vi "FlexMag - 23-03-2023.vi"() -> ()   [LabVIEW 2018] (continued)
                          n16847 = Less Or Equal?(x=w21889, y=0.2) -> (x <= y?=w21887:bool)
                          n16848 = case shown="True" w21887 {
                            tunnel: [FALSE TRUE] -> w21891
                            frame False {
                              n16849 = Wait Until Next ms Multiple(millisecond multiple=u32 200) -> ()  [unwired: 1 out]
                            }
                            frame True {
                            }
                          }
                          n16850 = local read "ch3 pumpdown alg"() -> (w21896:bool)
                          n16851 = local read "abort ch3"() -> (w21894:bool)
                          n16852 = Not(x=w21896) -> (.not. x?=w21895:bool)
                          n16853 = Compound Arithmetic op=OR(w21891, w21894, w21895) -> (w21897:bool)
                        }
                      }
                      frame True {
                      }
                    }
                  }
                }
              }
              frame #31 {
                # "tp start"
                n16854 = local read "ch3 pumpdown alg"() -> (w21903:bool)
                n16855 = case shown="True" w21903 {
                  frame False {
                  }
                  frame True {
                    n16856 = local read "abort ch3"() -> (w21904:bool)
                    n16857 = case shown="False" w21904 {
                      frame False {
                        n16858 = stacked-sequence {
                          frame #0 {
                            n16859 = flat-sequence {
                              frame #0 {
                                n16860 = local write "Tp3 auto start"(TRUE ("Tp1 auto start")) -> ()
                                n16861 = Wait (ms)(milliseconds to wait=u32 100) -> ()  [unwired: 1 out]
                              }
                              frame #1 {
                                n16862 = Wait (ms)(milliseconds to wait=u32 2000) -> ()  [unwired: 1 out]
                              }
                              frame #2 {
                                n16863 = disable-structure shown="Disabled" {
                                frame Disabled {
                                n16864 = local write "Tp1 Start initial"(TRUE ("Tp1 Start initial")) -> ()
                                }
                                frame Enabled {
                                }
                                }
                              }
                              frame #3 {
                                n16865 = Wait (ms)(milliseconds to wait=u32 2000) -> ()  [unwired: 1 out]
                              }
                              frame #4 {
                                n16866 = local write "Tp3 auto low speed"(TRUE ("Tp1 auto start")) -> ()
                                n16867 = Wait (ms)(milliseconds to wait=u32 100) -> ()  [unwired: 1 out]
                              }
                            }
                          }
                          frame #1 {
                            n16868 = while {
                              i -> [w21920]
                              stop <- w21914 stop-if-true
                              # "200 sec ?"
                              n16869 = Greater Or Equal?(x=w21920, y=1000) -> (x >= y?=w21913:bool)
                              n16870 = case shown="True" w21913 {
                                frame False {
                                }
                                frame True {
                                n16871 = local write "Warning Message"("CH3 PumpDown process  is canceled !\nCH3 TP couldn't be started" ("Warning Message")) -> ()
                                n16872 = local write "ch3 pumpdown error"(TRUE ("ch1 pumpdown error")) -> ()
                                }
                              }
                              n16873 = local read "ch3 pumpdown alg"() -> (w21917:bool)
                              n16874 = local read "ch3_tp_gui"() -> (w21912:bool)
                              n16875 = local read "abort ch3"() -> (w21915:bool)
                              n16876 = Not(x=w21917) -> (.not. x?=w21916:bool)
                              n16877 = Wait Until Next ms Multiple(millisecond multiple=u32 200) -> ()  [unwired: 1 out]
                              n16878 = Compound Arithmetic op=OR(w21912, w21915, w21916) -> (w21914:bool)
                            }
                          }
                        }
                      }
                      frame True {
                      }
                    }
                  }
                }
              }
              frame #32 {
                n16879 = local read "ch3 pumpdown alg"() -> (w21923:bool)
                n16880 = case shown="True" w21923 {
                  frame False {
                  }
                  frame True {
                    n16881 = local read "abort ch3"() -> (w21924:bool)
                    n16882 = case shown="False" w21924 {
                      frame False {
                        n16883 = local write "ch3 tp start led"(TRUE ("ch1 tp start led")) -> ()
                        n16884 = Wait (ms)(milliseconds to wait=u32 1000) -> ()  [unwired: 1 out]
                      }
                      frame True {
                      }
                    }
                  }
                }
              }
              frame #33 {
                n16885 = local read "ch3 pumpdown alg"() -> (w21927:bool)
                n16886 = case shown="True" w21927 {
                  frame False {
                  }
                  frame True {
                    n16887 = local read "abort ch3"() -> (w21928:bool)
                    n16888 = case shown="False" w21928 {
                      frame False {
                        n16889 = while {
                          i -> [w21935]
                          stop <- w21939 stop-if-true
                          # "30 min"
                          n16890 = Greater?(x=w21935, y=9000) -> (0:w21932:bool)
                          n16891 = case shown="True" w21932 {
                            frame False {
                            }
                            frame True {
                              n16892 = local write "Warning Message"("CH3 PumpDown process  is canceled !\nCH3 CH Pressure couldn't reach under 0.01 Torr" ("Warning Message")) -> ()
                              n16893 = local write "ch3 pumpdown error"(TRUE ("ch1 pumpdown error")) -> ()
                            }
                          }
                          n16894 = local read "ch3 ch pg torr"() -> (w21931:dbl)
                          n16895 = Less Or Equal?(x=w21931, y=0.09) -> (x <= y?=w21929:bool)
                          n16896 = case shown="False" w21929 {
                            tunnel: [FALSE TRUE] -> w21933
                            frame False {
                              n16897 = Wait Until Next ms Multiple(millisecond multiple=u32 200) -> ()  [unwired: 1 out]
                            }
                            frame True {
                            }
                          }
                          n16898 = local read "ch3 pumpdown alg"() -> (w21938:bool)
                          n16899 = local read "abort ch3"() -> (w21936:bool)
                          n16900 = Not(x=w21938) -> (.not. x?=w21937:bool)
                          n16901 = Compound Arithmetic op=OR(w21933, w21936, w21937) -> (w21939:bool)
                        }
                      }
                      frame True {
                      }
                    }
                  }
                }
              }
              frame #34 {
                n16902 = local read "ch3 pumpdown alg"() -> (w21945:bool)
                n16903 = case shown="True" w21945 {
                  frame False {
                  }
                  frame True {
                    n16904 = local read "abort ch3"() -> (w21946:bool)
                    n16905 = case shown="False" w21946 {
                      frame False {
                        n16906 = local write "ch3 ch press under 0.01 T led"(TRUE ("ch1 pressure under 0.05 torr led")) -> ()
                        n16907 = Wait (ms)(milliseconds to wait=u32 1000) -> ()  [unwired: 1 out]
                      }
                      frame True {
                      }
                    }
                  }
                }
              }
              frame #35 {
                n16908 = local read "ch3 pumpdown alg"() -> (w21949:bool)
                n16909 = case shown="True" w21949 {
                  frame False {
                  }
                  frame True {
                    n16910 = local read "abort ch3"() -> (w21950:bool)
                    n16911 = case shown="False" w21950 {
                      frame False {
                        n16912 = stacked-sequence {
                          frame #0 {
                            n16913 = while {
                              i -> [w21955]
                              stop <- w21959 stop-if-true
                              n16914 = Greater?(x=w21955, y=200) -> (0:w21952:bool)
                              n16915 = case shown="True" w21952 {
                                frame False {
                                }
                                frame True {
                                n16916 = local write "Warning Message"("CH3 PumpDown process  is canceled !\nCH3 CC couldn't be opened" ("Warning Message")) -> ()
                                n16917 = local write "ch3 pumpdown error"(TRUE ("ch1 pumpdown error")) -> ()
                                }
                              }
                              n16918 = local read "CH3_CC_DI"() -> (w21951:bool)
                              n16919 = case shown="False" w21951 {
                                tunnel: [FALSE TRUE] -> w21953
                                frame False {
                                n16920 = Wait Until Next ms Multiple(millisecond multiple=u32 200) -> ()  [unwired: 1 out]
                                n16921 = local write "CH3_CC_DO"(TRUE ("CH1_CC_DO")) -> ()
                                }
                                frame True {
                                }
                              }
                              n16922 = local read "ch3 pumpdown alg"() -> (w21958:bool)
                              n16923 = local read "abort ch3"() -> (w21956:bool)
                              n16924 = Not(x=w21958) -> (.not. x?=w21957:bool)
                              n16925 = Compound Arithmetic op=OR(w21953, w21956, w21957) -> (w21959:bool)
                            }
                          }
                          frame #1 {
                            n16926 = while {
                              i -> [w21968]
                              stop <- w21970 stop-if-true
                              n16927 = local read "ch3 pumpdown alg"() -> (w21971:bool)
                              n16928 = local read "abort ch3"() -> (w21973:bool)
                              n16929 = Greater Or Equal?(x=w21968, y=300) -> (x >= y?=w21966:bool)
                              n16930 = Not(x=w21971) -> (.not. x?=w21972:bool)
                              n16931 = Compound Arithmetic op=OR(w21966, w21973, w21972) -> (w21970:bool)
                              n16932 = Wait Until Next ms Multiple(millisecond multiple=u32 200) -> ()  [unwired: 1 out]
                            }
                          }
                        }
                      }
                      frame True {
                      }
                    }
                  }
                }
              }
              frame #36 {
                n16933 = local read "ch3 pumpdown alg"() -> (w21974:bool)
                n16934 = case shown="True" w21974 {
                  frame False {
                  }
                  frame True {
                    n16935 = local read "abort ch3"() -> (w21975:bool)
                    n16936 = case shown="False" w21975 {
                      frame False {
                        n16937 = local write "ch3 cc open led"(TRUE ("ch1 ch cc open led")) -> ()
                        n16938 = Wait (ms)(milliseconds to wait=u32 1000) -> ()  [unwired: 1 out]
                      }
                      frame True {
                      }
                    }
                  }
                }
              }
              frame #37 {
                n16939 = local read "ch3 pumpdown alg"() -> (w21978:bool)
                n16940 = case shown="True" w21978 {
                  frame False {
                  }
                  frame True {
                    n16941 = local read "abort ch3"() -> (w21979:bool)
                    n16942 = case shown="False" w21979 {
                      frame False {
                        n16943 = while {
                          i -> [w21990]
                          stop <- w21994 stop-if-true
                          # "60 min"
                          n16944 = Multiply(x=27000 ("y"), y=3) -> (x*y=w21980:i32)
                          n16945 = Greater?(x=w21990, y=w21980) -> (0:w21988:bool)
                          n16946 = case shown="True" w21988 {
                            frame False {
                            }
                            frame True {
                              n16947 = local write "Warning Message"("CH3 PumpDown process  is canceled !\nCH3 CH Pressure couldn't reach to desired pressure" ("Warning Message")) -> ()
                              n16948 = local write "ch3 pumpdown error"(TRUE ("ch1 pumpdown error")) -> ()
                            }
                          }
                          n16949 = local read "ch3 cc torr"() -> (w21987:dbl)
                          n16950 = Multiply(x=0.75, y="ch3 desired pressure") -> (x*y=w21983:dbl)
                          n16951 = Less Or Equal?(x=w21987, y=w21983) -> (x <= y?=w21986:bool)
                          n16952 = case shown="True" w21986 {
                            tunnel: [FALSE TRUE] -> w21989
                            frame False {
                              n16953 = Wait Until Next ms Multiple(millisecond multiple=u32 200) -> ()  [unwired: 1 out]
                            }
                            frame True {
                            }
                          }
                          n16954 = local read "ch3 pumpdown alg"() -> (w21993:bool)
                          n16955 = local read "abort ch3"() -> (w21991:bool)
                          n16956 = Not(x=w21993) -> (.not. x?=w21992:bool)
                          n16957 = Compound Arithmetic op=OR(w21989, w21991, w21992) -> (w21994:bool)
                        }
                      }
                      frame True {
                      }
                    }
                  }
                }
              }
              frame #38 {
                n16958 = local read "ch3 pumpdown alg"() -> (w22000:bool)
                n16959 = case shown="True" w22000 {
                  frame False {
                  }
                  frame True {
                    n16960 = local read "abort ch3"() -> (w22001:bool)
                    n16961 = case shown="False" w22001 {
                      frame False {
                        n16962 = local write "ch3 desired pressure led"(TRUE ("ch1 pumdown completed led")) -> ()
                        n16963 = Wait (ms)(milliseconds to wait=u32 1000) -> ()  [unwired: 1 out]
                      }
                      frame True {
                      }
                    }
                  }
                }
              }
              frame #39 {
                n16964 = local read "ch3 pumpdown alg"() -> (w22004:bool)
                n16965 = case shown="True" w22004 {
                  frame False {
                  }
                  frame True {
                    n16966 = local read "abort ch3"() -> (w22005:bool)
                    n16967 = case shown="False" w22005 {
                      frame False {
                        w22007 = TRUE ("Buzzer DO")
                        n16968 = local write "Buzzer DO"(w22007) -> ()
                        n16969 = local write "ch3 pd completed led"(w22007) -> ()
                        n16970 = Wait (ms)(milliseconds to wait=u32 3000) -> ()  [unwired: 1 out]
                        n16971 = local write "CH3_BG_BV_DO"(TRUE ("CH1_BG_BV_DO")) -> ()
                        n16972 = local write "System Status"("CH3 PUMPDOWN PROCESS COMPLETED" ("System Status")) -> ()
                      }
                      frame True {
                      }
                    }
                  }
                }
              }
              frame #40 {
                n16973 = local read "ch3 pumpdown alg"() -> (w22010:bool)
                n16974 = case shown="True" w22010 {
                  frame False {
                  }
                  frame True {
                    n16975 = local read "abort ch3"() -> (w22011:bool)
                    n16976 = case shown="False" w22011 {
                      frame False {
                        w22013 = FALSE ("Buzzer DO")
                        n16977 = local write "Buzzer DO"(w22013) -> ()
                        n16978 = local write "ch3 pumpdown alg"(w22013) -> ()
                        n16979 = local write "Pump Down CH3"(w22013) -> ()
                        n16980 = Wait (ms)(milliseconds to wait=u32 3000) -> ()  [unwired: 1 out]
                        n16981 = local write "System Status"("SEMI-AUTOMATIC MODE " ("System Status")) -> ()
                      }
                      frame True {
                      }
                    }
                  }
                }
              }
            }
          }
          frame True {
          }
        }
      }
    }
    n16982 = case shown="True" "ch3 shutdown alg" {
      frame False {
      }
      frame True {
        n16983 = local read "abort ch3"() -> (w21094:bool)
        n16984 = case shown="False" w21094 {
          frame False {
            n16985 = stacked-sequence {
              frame #0 {
                n16986 = stacked-sequence {
                  frame #0 {
                    n16987 = local write "ch3 vent?"(FALSE ("ch1 vent?")) -> ()
                    n16988 = Wait (ms)(milliseconds to wait=u32 1000) -> ()  [unwired: 1 out]
                  }
                  frame #1 {
                    n16989 = local write "System Status"("CH3 SHUTDOWN PROCESS IN PROGRESS" ("System Status")) -> ()
                  }
                  frame #2 {
                    n16990 = Two Button Dialog(message="Do you want to Vent CH3 ?", 1:"No, SHUTDOWN only" ("F button name (\"Cancel\")"), 2:"Yes, VENT! CH3" ("T button name (\"OK\")")) -> (T button?=w21098:bool)
                    "ch3 vent?" <- w21098
                    n16991 = case shown="True" w21098 {
                      frame False {
                      }
                      frame True {
                        w21102 = FALSE ("CH2_Trns_BP_Right_DO")
                        n16992 = local write "CH2_Trns_BP_Left_DO"(w21102) -> ()
                        n16993 = local write "CH4_Trns_BP_Right_DO"(w21102) -> ()
                      }
                    }
                  }
                }
              }
              frame #1 {
                # "ATMs close"
                n16994 = local read "ch3 shutdown alg"() -> (w21103:bool)
                n16995 = case shown="True" w21103 {
                  frame False {
                  }
                  frame True {
                    n16996 = local read "abort ch3"() -> (w21104:bool)
                    n16997 = case shown="False" w21104 {
                      frame False {
                        w21105 = FALSE ("CH1_PL_ATM_DO")
                        n16998 = local write "CH3_PL_ATM_DO"(w21105) -> ()
                        n16999 = local write "CH3_CH_ATM_DO"(w21105) -> ()
                        n17000 = Wait (ms)(milliseconds to wait=u32 3000) -> ()  [unwired: 1 out]
                      }
                      frame True {
                      }
                    }
                  }
                }
              }
              frame #2 {
                n17001 = local read "ch3 shutdown alg"() -> (w21107:bool)
                n17002 = case shown="True" w21107 {
                  frame False {
                  }
                  frame True {
                    n17003 = local read "abort ch3"() -> (w21108:bool)
                    n17004 = case shown="False" w21108 {
                      frame False {
                        n17005 = local write "ch3 sd atms close led"(TRUE ("ch1 sd cc close led")) -> ()
                        n17006 = Wait (ms)(milliseconds to wait=u32 1000) -> ()  [unwired: 1 out]
                      }
                      frame True {
                      }
                    }
                  }
                }
              }
              frame #3 {
                # "CC close"
                n17007 = local read "ch3 shutdown alg"() -> (w21111:bool)
                n17008 = case shown="True" w21111 {
                  frame False {
                  }
                  frame True {
                    n17009 = local read "abort ch3"() -> (w21112:bool)
                    n17010 = case shown="False" w21112 {
                      frame False {
                        n17011 = while {
                          i -> [w21117]
                          stop <- w21121 stop-if-true
                          n17012 = Greater?(x=w21117, y=100) -> (0:w21114:bool)
                          n17013 = case shown="True" w21114 {
                            frame False {
                            }
                            frame True {
                              n17014 = local write "Warning Message"("CH3 ShutDown process  is canceled !\nCH3 CC couldn't be closed" ("Warning Message")) -> ()
                              n17015 = local write "ch3 shutdown error"(TRUE ("ch1 pumpdown error")) -> ()
                            }
                          }
                          n17016 = local read "CH3_CC_DI"() -> (w21113:bool)
                          n17017 = case shown="True" w21113 {
                            tunnel: [TRUE FALSE] -> w21115
                            frame False {
                            }
                            frame True {
                              n17018 = Wait Until Next ms Multiple(millisecond multiple=u32 200) -> ()  [unwired: 1 out]
                              n17019 = local write "CH3_CC_DO"(FALSE ("CH1_CC_DO")) -> ()
                            }
                          }
                          n17020 = local read "ch3 shutdown alg"() -> (w21120:bool)
                          n17021 = local read "abort ch3"() -> (w21118:bool)
                          n17022 = Not(x=w21120) -> (.not. x?=w21119:bool)
                          n17023 = Compound Arithmetic op=OR(w21115, w21118, w21119) -> (w21121:bool)
                        }
                      }
                      frame True {
                      }
                    }
                  }
                }
              }
              frame #4 {
                n17024 = local read "ch3 shutdown alg"() -> (w21128:bool)
                n17025 = case shown="True" w21128 {
                  frame False {
                  }
                  frame True {
                    n17026 = local read "abort ch3"() -> (w21129:bool)
                    n17027 = case shown="False" w21129 {
                      frame False {
                        n17028 = local write "ch3 sd cc close led"(TRUE ("ch1 sd cc close led")) -> ()
                        n17029 = Wait (ms)(milliseconds to wait=u32 1000) -> ()  [unwired: 1 out]
                      }
                      frame True {
                      }
                    }
                  }
                }
              }
              frame #5 {
                # "bg bv close"
                n17030 = local read "ch3 shutdown alg"() -> (w21132:bool)
                n17031 = case shown="True" w21132 {
                  frame False {
                  }
                  frame True {
                    n17032 = local read "abort ch3"() -> (w21133:bool)
                    n17033 = case shown="False" w21133 {
                      frame False {
                        n17034 = while {
                          i -> [w21138]
                          stop <- w21142 stop-if-true
                          n17035 = Greater?(x=w21138, y=100) -> (0:w21135:bool)
                          n17036 = case shown="True" w21135 {
                            frame False {
                            }
                            frame True {
                              n17037 = local write "Warning Message"("CH3 ShutDown process  is canceled !\nCH3 BG BV couldn't be closed" ("Warning Message")) -> ()
                              n17038 = local write "ch3 shutdown error"(TRUE ("ch1 pumpdown error")) -> ()
                            }
                          }
                          n17039 = local read "CH3_BG_BV_DI"() -> (w21134:bool)
                          n17040 = case shown="True" w21134 {
                            tunnel: [TRUE FALSE] -> w21136
                            frame False {
                            }
                            frame True {
                              n17041 = Wait Until Next ms Multiple(millisecond multiple=u32 200) -> ()  [unwired: 1 out]
                              n17042 = local write "CH3_BG_BV_DO"(FALSE ("CH1_CC_DO")) -> ()
                            }
                          }
                          n17043 = local read "ch3 shutdown alg"() -> (w21141:bool)
                          n17044 = local read "abort ch3"() -> (w21139:bool)
                          n17045 = Not(x=w21141) -> (.not. x?=w21140:bool)
                          n17046 = Compound Arithmetic op=OR(w21136, w21139, w21140) -> (w21142:bool)
                        }
                      }
                      frame True {
                      }
                    }
                  }
                }
              }
              frame #6 {
                n17047 = local read "ch3 shutdown alg"() -> (w21149:bool)
                n17048 = case shown="True" w21149 {
                  frame False {
                  }
                  frame True {
                    n17049 = local read "abort ch3"() -> (w21150:bool)
                    n17050 = case shown="False" w21150 {
                      frame False {
                        n17051 = local write "ch3 sd bg bv close led"(TRUE ("ch1 sd cc close led")) -> ()
                        n17052 = Wait (ms)(milliseconds to wait=u32 1000) -> ()  [unwired: 1 out]
                      }
                      frame True {
                      }
                    }
                  }
                }
              }
              frame #7 {
                # "TP stop"
                n17053 = local read "ch3 shutdown alg"() -> (w21153:bool)
                n17054 = case shown="True" w21153 {
                  frame False {
                  }
                  frame True {
                    n17055 = local read "abort ch3"() -> (w21154:bool)
                    n17056 = case shown="False" w21154 {
                      frame False {
                        n17057 = stacked-sequence {
                          frame #0 {
                            n17058 = flat-sequence {
                              frame #0 {
                                n17059 = local write "Tp3 auto stop"(TRUE ("Tp1 auto stop")) -> ()
                                n17060 = Wait (ms)(milliseconds to wait=u32 100) -> ()  [unwired: 1 out]
                              }
                              frame #1 {
                                n17061 = Wait (ms)(milliseconds to wait=u32 5000) -> ()  [unwired: 1 out]
                              }
                              frame #2 {
                                n17062 = local write "Tp3 auto stop"(TRUE ("Tp1 auto stop")) -> ()
                                n17063 = Wait (ms)(milliseconds to wait=u32 100) -> ()  [unwired: 1 out]
                              }
                            }
                          }
                          frame #1 {
                            n17064 = while {
                              i -> [w21171]
                              stop <- w21166 stop-if-true
                              n17065 = Multiply(x=3000 ("y"), y=5) -> (x*y=w21161:i32)
                              n17066 = Greater Or Equal?(x=w21171, y=w21161) -> (x >= y?=w21165:bool)
                              n17067 = case shown="True" w21165 {
                                frame False {
                                }
                                frame True {
                                n17068 = local write "Warning Message"("CH3 ShutDown process  is canceled !\nCH3 TP couldn't be stopped" ("Warning Message")) -> ()
                                n17069 = local write "ch3 shutdown error"(TRUE ("ch1 pumpdown error")) -> ()
                                }
                              }
                              n17070 = local read "ch3 shutdown alg"() -> (w21169:bool)
                              n17071 = local read "ch3_tp_gui"() -> (w21164:bool)
                              n17072 = local read "abort ch3"() -> (w21167:bool)
                              n17073 = Not(x=w21164) -> (.not. x?=w21163:bool)
                              n17074 = Not(x=w21169) -> (.not. x?=w21168:bool)
                              n17075 = Wait Until Next ms Multiple(millisecond multiple=u32 200) -> ()  [unwired: 1 out]
                              n17076 = Compound Arithmetic op=OR(w21163, w21167, w21168) -> (w21166:bool)
                            }
                          }
                        }
                      }
                      frame True {
                      }
                    }
                  }
                }
              }
              frame #8 {
                n17077 = local read "ch3 shutdown alg"() -> (w21174:bool)
                n17078 = case shown="True" w21174 {
                  frame False {
                  }
                  frame True {
                    n17079 = local read "abort ch3"() -> (w21175:bool)
                    n17080 = case shown="False" w21175 {
                      frame False {
                        n17081 = local write "ch3 sd tp stop led"(TRUE ("ch1 sd cc close led")) -> ()
                        n17082 = Wait (ms)(milliseconds to wait=u32 1000) -> ()  [unwired: 1 out]
                      }
                      frame True {
                      }
                    }
                  }
                }
              }
              frame #9 {
                # "tp bv close"
                n17083 = local read "ch3 shutdown alg"() -> (w21178:bool)
                n17084 = case shown="True" w21178 {
                  frame False {
                  }
                  frame True {
                    n17085 = local read "abort ch3"() -> (w21179:bool)
                    n17086 = case shown="False" w21179 {
                      frame False {
                        n17087 = while {
                          i -> [w21184]
                          stop <- w21188 stop-if-true
                          n17088 = Greater?(x=w21184, y=100) -> (0:w21181:bool)
                          n17089 = case shown="True" w21181 {
                            frame False {
                            }
                            frame True {
                              n17090 = local write "Warning Message"("CH3 ShutDown process  is canceled !\nCH3 TP BV couldn't be closed" ("Warning Message")) -> ()
                              n17091 = local write "ch3 shutdown error"(TRUE ("ch1 pumpdown error")) -> ()
                            }
                          }
                          n17092 = local read "CH3_TP_BV_DI"() -> (w21180:bool)
                          n17093 = case shown="True" w21180 {
                            tunnel: [TRUE FALSE] -> w21182
                            frame False {
                            }
                            frame True {
                              n17094 = Wait Until Next ms Multiple(millisecond multiple=u32 200) -> ()  [unwired: 1 out]
                              n17095 = local write "CH3_TP_BV_DO"(FALSE ("CH1_CC_DO")) -> ()
                            }
                          }
                          n17096 = local read "ch3 shutdown alg"() -> (w21187:bool)
                          n17097 = local read "abort ch3"() -> (w21185:bool)
                          n17098 = Not(x=w21187) -> (.not. x?=w21186:bool)
                          n17099 = Compound Arithmetic op=OR(w21182, w21185, w21186) -> (w21188:bool)
                        }
                      }
                      frame True {
                      }
                    }
                  }
                }
              }
              frame #10 {
                n17100 = local read "ch3 shutdown alg"() -> (w21195:bool)
                n17101 = case shown="True" w21195 {
                  frame False {
                  }
                  frame True {
                    n17102 = local read "abort ch3"() -> (w21196:bool)
                    n17103 = case shown="False" w21196 {
                      frame False {
                        n17104 = local write "ch3 sd tp bv close led"(TRUE ("ch1 sd cc close led")) -> ()
                        n17105 = Wait (ms)(milliseconds to wait=u32 1000) -> ()  [unwired: 1 out]
                      }
                      frame True {
                      }
                    }
                  }
                }
              }
              frame #11 {
                # "mp stop"
                n17106 = local read "ch3 shutdown alg"() -> (w21199:bool)
                n17107 = case shown="True" w21199 {
                  frame False {
                  }
                  frame True {
                    n17108 = local read "abort ch3"() -> (w21200:bool)
                    n17109 = case shown="False" w21200 {
                      frame False {
                        n17110 = while {
                          i -> [w21205]
                          stop <- w21209 stop-if-true
                          n17111 = Greater?(x=w21205, y=100) -> (0:w21202:bool)
                          n17112 = case shown="True" w21202 {
                            frame False {
                            }
                            frame True {
                              n17113 = local write "Warning Message"("CH3 ShutDown process  is canceled !\nCH3 MP couldn't be stopped" ("Warning Message")) -> ()
                              n17114 = local write "ch3 shutdown error"(TRUE ("ch1 pumpdown error")) -> ()
                            }
                          }
                          n17115 = local read "CH3_MP_DI"() -> (w21201:bool)
                          n17116 = case shown="True" w21201 {
                            tunnel: [TRUE FALSE] -> w21203
                            frame False {
                            }
                            frame True {
                              n17117 = Wait Until Next ms Multiple(millisecond multiple=u32 200) -> ()  [unwired: 1 out]
                              n17118 = local write "CH3_MP_DO"(FALSE ("CH1_CC_DO")) -> ()
                            }
                          }
                          n17119 = local read "ch3 shutdown alg"() -> (w21208:bool)
                          n17120 = local read "abort ch3"() -> (w21206:bool)
                          n17121 = Not(x=w21208) -> (.not. x?=w21207:bool)
                          n17122 = Compound Arithmetic op=OR(w21203, w21206, w21207) -> (w21209:bool)
                        }
                      }
                      frame True {
                      }
                    }
                  }
                }
              }
              frame #12 {
                n17123 = local read "ch3 shutdown alg"() -> (w21216:bool)
                n17124 = case shown="True" w21216 {
                  frame False {
                  }
                  frame True {
                    n17125 = local read "abort ch3"() -> (w21217:bool)
                    n17126 = case shown="False" w21217 {
                      frame False {
                        n17127 = local write "ch3 sd mp stop led"(TRUE ("ch1 sd cc close led")) -> ()
                        n17128 = Wait (ms)(milliseconds to wait=u32 1000) -> ()  [unwired: 1 out]
                      }
                      frame True {
                      }
                    }
                  }
                }
              }
              frame #13 {
                # "pl vbv open"
                n17129 = local read "ch3 shutdown alg"() -> (w21220:bool)
                n17130 = case shown="True" w21220 {
                  frame False {
                  }
                  frame True {
                    n17131 = local read "abort ch3"() -> (w21221:bool)
                    n17132 = case shown="False" w21221 {
                      frame False {
                        n17133 = while {
                          i -> [w21226]
                          stop <- w21230 stop-if-true
                          n17134 = Greater?(x=w21226, y=100) -> (0:w21223:bool)
                          n17135 = case shown="True" w21223 {
                            frame False {
                            }
                            frame True {
                              n17136 = local write "Warning Message"("CH3 ShutDown process  is canceled !\nCH3 PL VBV couldn't be opened" ("Warning Message")) -> ()
                              n17137 = local write "ch3 shutdown alg"(TRUE ("ch1 pumpdown error")) -> ()
                            }
                          }
                          n17138 = local read "CH3_PL_VBV_DI"() -> (w21222:bool)
                          n17139 = case shown="False" w21222 {
                            tunnel: [FALSE TRUE] -> w21224
                            frame False {
                              n17140 = Wait Until Next ms Multiple(millisecond multiple=u32 200) -> ()  [unwired: 1 out]
                              n17141 = local write "CH3_PL_VBV_DO"(TRUE ("CH1_CC_DO")) -> ()
                            }
                            frame True {
                            }
                          }
                          n17142 = local read "ch3 shutdown alg"() -> (w21229:bool)
                          n17143 = local read "abort ch3"() -> (w21227:bool)
                          n17144 = Not(x=w21229) -> (.not. x?=w21228:bool)
                          n17145 = Compound Arithmetic op=OR(w21224, w21227, w21228) -> (w21230:bool)
                        }
                      }
                      frame True {
                      }
                    }
                  }
                }
              }
              frame #14 {
                n17146 = local read "ch3 shutdown alg"() -> (w21237:bool)
                n17147 = case shown="True" w21237 {
                  frame False {
                  }
                  frame True {
                    n17148 = local read "abort ch3"() -> (w21238:bool)
                    n17149 = case shown="False" w21238 {
                      frame False {
                        n17150 = local write "ch3 sd pl vbv open led"(TRUE ("ch1 sd cc close led")) -> ()
                        n17151 = Wait (ms)(milliseconds to wait=u32 1000) -> ()  [unwired: 1 out]
                      }
                      frame True {
                      }
                    }
                  }
                }
              }
              frame #15 {
                n17152 = local read "ch3 shutdown alg"() -> (w21241:bool)
                n17153 = case shown="True" w21241 {
                  frame False {
                  }
                  frame True {
                    n17154 = local read "abort ch3"() -> (w21242:bool)
                    n17155 = case shown="False" w21242 {
                      frame False {
                        n17156 = local read "ch3 vent?"() -> (w21243:bool)
                        n17157 = case shown="False" w21243 {
                          frame False {
                            n17158 = stacked-sequence {
                              frame #0 {
                                n17159 = local read "ch3 shutdown alg"() -> (w21244:bool)
                                n17160 = case shown="True" w21244 {
                                frame False {
                                }
                                frame True {
                                n17161 = flat-sequence {
                                frame #0 {
                                n17162 = local write "pcgv3 auto close"(TRUE ("pcgv1 auto open")) -> ()
                                }
                                frame #1 {
                                n17163 = Wait (ms)(milliseconds to wait=u32 2000) -> ()  [unwired: 1 out]
                                }
                                frame #2 {
                                n17164 = local write "pcgv3 auto close"(TRUE ("pcgv1 auto open")) -> ()
                                }
                                }
                                }
                                }
                              }
                              frame #1 {
                                n17165 = while {
                                i -> [w21255]
                                stop <- w21251 stop-if-true
                                n17166 = Greater Or Equal?(x=w21255, y=200) -> (x >= y?=w21257:bool)
                                n17167 = case shown="True" w21257 {
                                frame False {
                                }
                                frame True {
                                n17168 = local write "ch3 shutdown error"(TRUE ("ch1 pumpdown error")) -> ()
                                n17169 = local write "Warning Message"("CH3 ShutDown process  is canceled !\nCH3 PC GV couldn't be closed" ("Warning Message")) -> ()
                                }
                                }
                                n17170 = local read "ch3_pcgv_gui"() -> (w21248:bool)
                                n17171 = local read "abort ch3"() -> (w21252:bool)
                                n17172 = local read "ch3 shutdown alg"() -> (w21254:bool)
                                n17173 = Wait Until Next ms Multiple(millisecond multiple=u32 200) -> ()  [unwired: 1 out]
                                n17174 = Not(x=w21248) -> (.not. x?=w21249:bool)
                                n17175 = Not(x=w21254) -> (.not. x?=w21253:bool)
                                n17176 = Compound Arithmetic op=OR(w21249, w21252, w21253) -> (w21251:bool)
                                }
                              }
                            }
                          }
                          frame True {
                            n17177 = stacked-sequence {
                              frame #0 {
                                n17178 = local read "ch3 shutdown alg"() -> (w21260:bool)
                                n17179 = case shown="True" w21260 {
                                frame False {
                                }
                                frame True {
                                n17180 = flat-sequence {
                                frame #0 {
                                n17181 = local write "pcgv3 auto open"(TRUE ("pcgv1 auto open")) -> ()
                                }
                                frame #1 {
                                n17182 = Wait (ms)(milliseconds to wait=u32 2000) -> ()  [unwired: 1 out]
                                }
                                frame #2 {
                                n17183 = local write "pcgv3 auto open"(TRUE ("pcgv1 auto open")) -> ()
                                }
                                }
                                }
                                }
                              }
                              frame #1 {
                                n17184 = while {
                                i -> [w21270]
                                stop <- w21266 stop-if-true
                                n17185 = Greater Or Equal?(x=w21270, y=200) -> (x >= y?=w21272:bool)
                                n17186 = case shown="True" w21272 {
                                frame False {
                                }
                                frame True {
                                n17187 = local write "ch3 shutdown error"(TRUE ("ch1 pumpdown error")) -> ()
                                n17188 = local write "Warning Message"("CH3 ShutDown process  is canceled !\nCH3 PC GV couldn't be opened" ("Warning Message")) -> ()
                                }
                                }
                                n17189 = local read "ch3 shutdown alg"() -> (w21269:bool)
                                n17190 = local read "ch3_pcgv_gui"() -> (w21265:bool)
                                n17191 = local read "abort ch3"() -> (w21267:bool)
                                n17192 = Wait Until Next ms Multiple(millisecond multiple=u32 200) -> ()  [unwired: 1 out]
                                n17193 = Not(x=w21269) -> (.not. x?=w21268:bool)
                                n17194 = Compound Arithmetic op=OR(w21265, w21267, w21268) -> (w21266:bool)
                                }
                              }
                            }
                          }
                        }
                      }
                      frame True {
                      }
                    }
                  }
                }
              }
              frame #16 {
                n17195 = local read "ch3 shutdown alg"() -> (w21275:bool)
                n17196 = case shown="True" w21275 {
                  frame False {
                  }
                  frame True {
                    n17197 = local read "abort ch3"() -> (w21276:bool)
                    n17198 = case shown="False" w21276 {
                      frame False {
                        n17199 = local read "ch3 vent?"() -> (w21277:bool)
                        n17200 = case shown="False" w21277 {
                          frame False {
                            n17201 = local write "ch3 sd pcgv close led"(TRUE ("ch1 sd cc close led")) -> ()
                            n17202 = Wait (ms)(milliseconds to wait=u32 1000) -> ()  [unwired: 1 out]
                          }
                          frame True {
                            n17203 = local write "ch3 sd pcgv open led"(TRUE ("ch1 sd cc close led")) -> ()
                            n17204 = Wait (ms)(milliseconds to wait=u32 1000) -> ()  [unwired: 1 out]
                          }
                        }
                      }
                      frame True {
                      }
                    }
                  }
                }
              }
              frame #17 {
                n17205 = local read "ch3 shutdown alg"() -> (w21282:bool)
                n17206 = case shown="True" w21282 {
                  frame False {
                  }
                  frame True {
                    n17207 = local read "abort ch3"() -> (w21283:bool)
                    n17208 = case shown="False" w21283 {
                      frame False {
                        n17209 = local read "ch3 vent?"() -> (w21284:bool)
                        n17210 = case shown="True" w21284 {
                          frame False {
                            n17211 = while {
                              i -> [w21291]
                              stop <- w21287 stop-if-true
                              n17212 = Greater Or Equal?(x=w21291, y=100) -> (x >= y?=w21293:bool)
                              n17213 = case shown="True" w21293 {
                                frame False {
                                }
                                frame True {
                                n17214 = local write "ch3 shutdown error"(TRUE ("ch1 pumpdown error")) -> ()
                                n17215 = local write "Warning Message"("CH3 ShutDown process  is canceled !\nCH3 Trns BP Left couldn't be opened" ("Warning Message")) -> ()
                                }
                              }
                              n17216 = local read "CH3_Trns_BP_Left_DI"() -> (w21286:bool)
                              n17217 = case shown="False" w21286 {
                                tunnel: [FALSE TRUE] -> w21285
                                frame False {
                                n17218 = Wait Until Next ms Multiple(millisecond multiple=u32 200) -> ()  [unwired: 1 out]
                                n17219 = local write "CH3_Trns_BP_Left_DO"(FALSE ("CH1_WFC_DO")) -> ()
                                }
                                frame True {
                                }
                              }
                              n17220 = local read "ch3 shutdown alg"() -> (w21290:bool)
                              n17221 = local read "abort ch3"() -> (w21288:bool)
                              n17222 = Not(x=w21290) -> (.not. x?=w21289:bool)
                              n17223 = Compound Arithmetic op=OR(w21285, w21288, w21289) -> (w21287:bool)
                            }
                          }
                          frame True {
                            n17224 = local read "ch3_4 vacuum level"() -> (w21301:string)
                            n17225 = Equal?(x=w21301, y="VACUUM") -> (x = y?=w21300:bool)
                            n17226 = case shown="True" w21300 {
                              frame False {
                              }
                              frame True {
                                n17227 = while {
                                i -> [w21309]
                                stop <- w21305 stop-if-true
                                n17228 = Greater Or Equal?(x=w21309, y=200) -> (x >= y?=w21311:bool)
                                n17229 = case shown="True" w21311 {
                                frame False {
                                }
                                frame True {
                                n17230 = local write "ch3 shutdown error"(TRUE ("ch1 pumpdown error")) -> ()
                                n17231 = local write "Warning Message"("CH3 ShutDown process  is canceled !\nCH3 Trns BP Left couldn't be closed" ("Warning Message")) -> ()
                                }
                                }
                                n17232 = local read "CH3_Trns_BP_Left_DI"() -> (w21304:bool)
                                n17233 = case shown="False" w21304 {
                                tunnel: [FALSE TRUE] -> w21303
                                frame False {
                                n17234 = Wait Until Next ms Multiple(millisecond multiple=u32 200) -> ()  [unwired: 1 out]
                                n17235 = local write "CH3_Trns_BP_Left_DO"(TRUE ("CH1_WFC_DO")) -> ()
                                }
                                frame True {
                                }
                                }
                                n17236 = local read "abort ch3"() -> (w21306:bool)
                                n17237 = local read "ch3 shutdown alg"() -> (w21308:bool)
                                n17238 = Not(x=w21308) -> (.not. x?=w21307:bool)
                                n17239 = Compound Arithmetic op=OR(w21303, w21306, w21307) -> (w21305:bool)
                                }
                              }
                            }
                          }
                        }
                      }
                      frame True {
                      }
                    }
                  }
                }
              }
              frame #18 {
                n17240 = local read "ch3 shutdown alg"() -> (w21318:bool)
                n17241 = case shown="True" w21318 {
                  frame False {
                  }
                  frame True {
                    n17242 = local read "abort ch3"() -> (w21319:bool)
                    n17243 = case shown="False" w21319 {
                      frame False {
                        n17244 = local read "ch3 vent?"() -> (w21320:bool)
                        n17245 = case shown="False" w21320 {
                          frame False {
                            n17246 = local write "ch3 sd trns bp left close led"(TRUE ("ch1 sd cc close led")) -> ()
                            n17247 = Wait (ms)(milliseconds to wait=u32 1000) -> ()  [unwired: 1 out]
                          }
                          frame True {
                            n17248 = local write "ch3 sd trns bp left open led"(TRUE ("ch1 sd cc close led")) -> ()
                            n17249 = Wait (ms)(milliseconds to wait=u32 1000) -> ()  [unwired: 1 out]
                          }
                        }
                      }
                      frame True {
                      }
                    }
                  }
                }
              }
              frame #19 {
                n17250 = local read "ch3 shutdown alg"() -> (w21325:bool)
                n17251 = case shown="True" w21325 {
                  frame False {
                  }
                  frame True {
                    n17252 = local read "abort ch3"() -> (w21326:bool)
                    n17253 = case shown="False" w21326 {
                      frame False {
                        n17254 = local read "ch3 vent?"() -> (w21327:bool)
                        n17255 = case shown="True" w21327 {
                          frame False {
                            n17256 = while {
                              i -> [w21334]
                              stop <- w21330 stop-if-true
                              n17257 = Greater Or Equal?(x=w21334, y=200) -> (x >= y?=w21336:bool)
                              n17258 = case shown="True" w21336 {
                                frame False {
                                }
                                frame True {
                                n17259 = local write "ch3 shutdown error"(TRUE ("ch1 pumpdown error")) -> ()
                                n17260 = local write "Warning Message"("CH3 ShutDown process  is canceled !\nCH3 Trns BP Right couldn't be closed" ("Warning Message")) -> ()
                                }
                              }
                              n17261 = local read "CH3_Trns_BP_Right_DI"() -> (w21329:bool)
                              n17262 = case shown="True" w21329 {
                                tunnel: [TRUE FALSE] -> w21328
                                frame False {
                                }
                                frame True {
                                n17263 = Wait Until Next ms Multiple(millisecond multiple=u32 200) -> ()  [unwired: 1 out]
                                n17264 = local write "CH3_Trns_BP_Right_DO"(FALSE ("CH1_WFC_DO")) -> ()
                                }
                              }
                              n17265 = local read "abort ch3"() -> (w21331:bool)
                              n17266 = local read "ch3 shutdown alg"() -> (w21333:bool)
                              n17267 = Not(x=w21333) -> (.not. x?=w21332:bool)
                              n17268 = Compound Arithmetic op=OR(w21328, w21331, w21332) -> (w21330:bool)
                            }
                          }
                          frame True {
                            n17269 = local read "ch2_3 vacuum level"() -> (w21344:string)
                            n17270 = Equal?(x=w21344, y="VACUUM") -> (x = y?=w21343:bool)
                            n17271 = case shown="True" w21343 {
                              frame False {
                              }
                              frame True {
                                n17272 = while {
                                i -> [w21352]
                                stop <- w21348 stop-if-true
                                n17273 = Greater Or Equal?(x=w21352, y=100) -> (x >= y?=w21354:bool)
                                n17274 = case shown="True" w21354 {
                                frame False {
                                }
                                frame True {
                                n17275 = local write "ch3 shutdown error"(TRUE ("ch1 pumpdown error")) -> ()
                                n17276 = local write "Warning Message"("CH3 ShutDown process  is canceled !\nCH3 Trns BP Right couldn't be opened" ("Warning Message")) -> ()